vi "Remove IV curve offset.vi"() -> ()   [LabVIEW 2016]
panel:
  out "X closest to 0":dbl
  out "A vs B after offset":cluster{dbl[], dbl[]}[](graph)
  out "middle element X":dbl=0.0928822327027844
  out "size X":i32=9999
  out "Array Y":dbl[](array[numeric])
  out "Array X":dbl[](array[numeric])
  in  "A vs B":cluster{dbl[], dbl[]}[](graph)=[{array[9999 elements], array[9999 elements]}, {array[9999 elements], array[9999 elements]}, {array[9999 elements], array[9999 elements]}, {array[9999 elements], array[9999 elements]}, {array[9999 elements], array[9999 elements]}, {array[9999 elements], array[9999 elements]}, {array[9999 elements], array[9999 elements]}, {array[9999 elements], array[9999 elements]}, {array[9999 elements], array[9999 elements]}, {array[9999 elements], array[9999 elements]}, {array[9999 elements], array[9999 elements]}, {array[9999 elements], array[9999 elements]}, {array[9999 elements], array[9999 elements]}, {array[9999 elements], array[9999 elements]}]
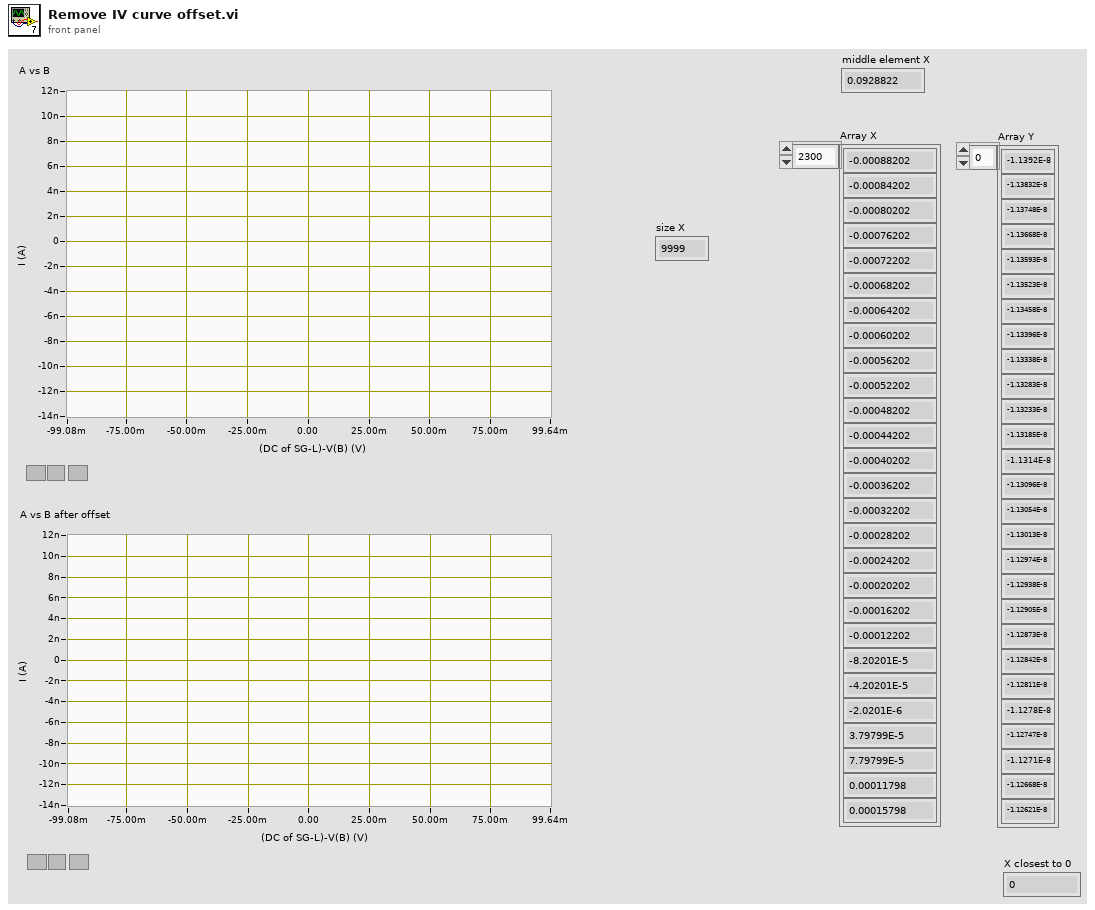
[diagram p1: front panel]
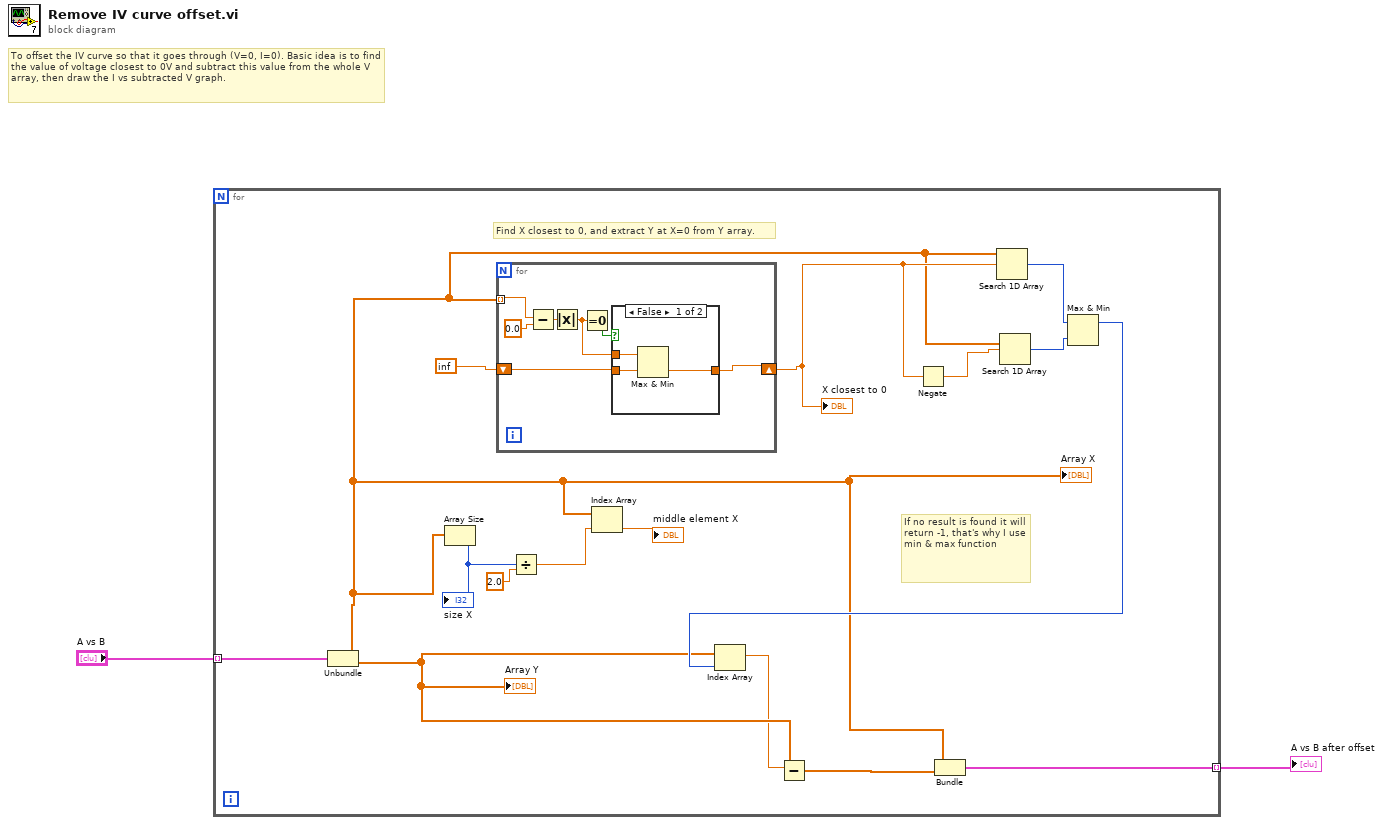
[diagram p0: block diagram]
diagram:
  # "To offset the IV curve so that it goes through (V=0, I=0). Basic idea is to find the value of voltage closest to 0V and subtract this value from the whole V array, then draw the I vs subtracted V graph."
  n1 = for {
    tunnel: "A vs B" -> [w18] mode=indexing
    tunnel: [w12] -> w1 mode=indexing
    # "Find X closest to 0, and extract Y at X=0 from Y array."
    # "If no result is found it will return -1, that's why I use min & max function"
    n2 = Unbundle(w18) -> (w4:dbl[], w5:dbl[])
    "Array X" <- w4
    "Array Y" <- w5
    n3 = Array Size(array=w4) -> (size(s)=w17:i32)
    "size X" <- w17
    n4 = for {
      tunnel: w4 -> [w20] mode=indexing
      shift-right: [w19] -> w10
      shift-left: inf -> [w25]
      n5 = Subtract(x=w20, y=0.0) -> (x-y=w23:dbl)
      n6 = Absolute Value(x=w23) -> (abs(x)=w21:dbl)
      n7 = Equal To 0?(x=w21) -> (x = 0?=w22:bool)
      n8 = case shown="False" w22 {
        tunnel: w25 -> [w28 _]
        tunnel: [w27 w29] -> w19
        tunnel: w21 -> [w26 w29]
        frame False {
          n9 = Max & Min(x=w26, y=w28) -> (min(x,y)=w27:dbl)  [unwired: 1 out]
        }
        frame True {
        }
      }
    }
    "X closest to 0" <- w10
    n10 = Divide(x=w17, y=2.0) -> (x/y=w14:dbl)
    n11 = Index Array(array=w4, index=w14) -> (element=→"middle element X":dbl)
    n12 = Negate(x=w10) -> (-x=w9:dbl)
    n13 = Search 1D Array(1D array=w4, element=w10) -> (index of element=w8:i32)  [unwired: 1 in]
    n14 = Search 1D Array(1D array=w4, element=w9) -> (index of element=w7:i32)  [unwired: 1 in]
    n15 = Max & Min(x=w8, y=w7) -> (max(x,y)=w6:i32)  [unwired: 1 out]
    n16 = Index Array(array=w5, index=w6) -> (element=w3:dbl)
    n17 = Subtract(x=w5, y=w3) -> (x-y=w13:dbl[])
    n18 = Bundle(w4, w13) -> (w12:cluster{dbl[], dbl[]})  [unwired: 1 in]
  }
  "A vs B after offset" <- w1
